vi "ATF_PUMP_PID_screen_V0.0.vi"() -> ()   [LabVIEW 2022 SP3]
panel:
  out "Countdown Timer (CDT)":dbl format="T%<+%H:%M:%S%3u>t"
  out "Date":timestamp format="%<%d/%m/%Y>T"
  in  "Close":bool
  in  "Screen No":dbl
  out "Indian Standard Time (IST)":timestamp format="%<%H:%M:%S%2u>T"
  out "B_AT_T_04":dbl format="%.2f bar"
  out "B_AT_T_05":dbl format="%.2f bar"
  out "B_ATP_P_01 76":dbl format="%.2f bar"
  out "B_ATP_P_01 75":dbl format="%.2f bar"
  out "B_ATP_P_01 74":dbl format="%.2f bar"
  out "B_ATP_P_01 73":dbl format="%.2f bar"
  out "B_ATP_P_01 72":dbl format="%.2f bar"
  out "B_ATP_P_01 71":dbl format="%.2f bar"
  out "B_ATP_P_01 70":dbl format="%.2f bar"
  out "B_ATP_P_01 69":dbl format="%.2f bar"
  out "B_ATP_P_01 68":dbl format="%.2f bar"
  out "B_ATP_P_01 67":dbl format="%.2f bar"
  out "B_ATP_P_01 66":dbl format="%.2f bar"
  out "B_ATP_P_01 65":dbl format="%.2f bar"
  out "B_ATP_P_01 64":dbl format="%.2f bar"
  out "B_ATP_P_01 63":dbl format="%.2f bar"
  out "B_ATP_P_01 62":dbl format="%.2f bar"
  out "B_ATP_P_01 61":dbl format="%.2f bar"
  out "B_ATP_P_01 60":dbl format="%.2f bar"
  out "B_ATP_P_01 59":dbl format="%.2f bar"
  out "B_ATP_P_01 58":dbl format="%.2f bar"
  out "B_ATP_P_01 57":dbl format="%.2f bar"
  out "B_ATP_P_01 56":dbl format="%.2f bar"
  out "B_ATP_P_01 55":dbl format="%.2f bar"
  out "B_ATP_P_01 54":dbl format="%.2f bar"
  out "B_ATP_P_01 53":dbl format="%.2f bar"
  out "B_ATP_P_01 52":dbl format="%.2f bar"
  out "B_ATP_P_01 51":dbl format="%.2f bar"
  out "B_ATP_P_01 50":dbl format="%.2f bar"
  out "B_ATP_P_01 49":dbl format="%.2f bar"
  out "B_ATP_P_01 48":dbl format="%.2f bar"
  out "B_ATP_P_01 47":dbl format="%.2f bar"
  out "B_ATP_P_01 46":dbl format="%.2f bar"
  out "B_ATP_P_01 45":dbl format="%.2f bar"
  out "B_ATP_P_01 44":dbl format="%.2f bar"
  out "B_ATP_P_01 43":dbl format="%.2f bar"
  out "B_ATP_P_01 42":dbl format="%.2f bar"
  out "B_ATP_P_01 41":dbl format="%.2f bar"
  out "B_ATP_P_01 40":dbl format="%.2f bar"
  out "B_ATP_P_01 39":dbl format="%.2f bar"
  out "B_ATP_P_01 38":dbl format="%.2f bar"
  out "B_ATP_P_01 37":dbl format="%.2f bar"
  out "B_ATP_P_01 36":dbl format="%.2f bar"
  out "B_ATP_P_01 35":dbl format="%.2f bar"
  out "B_ATP_P_01 34":dbl format="%.2f bar"
  out "B_ATP_P_01 33":dbl format="%.2f bar"
  out "B_ATP_P_01 32":dbl format="%.2f bar"
  out "B_ATP_P_01 31":dbl format="%.2f bar"
  out "B_ATP_P_01 30":dbl format="%.2f bar"
  out "B_ATP_P_01 29":dbl format="%.2f bar"
  out "B_ATP_P_01 28":dbl format="%.2f bar"
  out "B_ATP_P_01 27":dbl format="%.2f bar"
  out "B_ATP_P_01 26":dbl format="%.2f bar"
  out "B_ATP_P_01 25":dbl format="%.2f bar"
  out "B_ATP_P_01 24":dbl format="%.2f bar"
  out "B_ATP_P_01 23":dbl format="%.2f bar"
  out "B_ATP_P_01 22":dbl format="%.2f bar"
  out "B_ATP_P_01 21":dbl format="%.2f bar"
  out "B_ATP_P_01 20":dbl format="%.2f bar"
  out "B_ATP_P_01 19":dbl format="%.2f bar"
  out "B_ATP_P_01 18":dbl format="%.2f bar"
  out "B_ATP_P_01 17":dbl format="%.2f bar"
  out "B_ATP_P_01 16":dbl format="%.2f bar"
  out "B_ATP_P_01 15":dbl format="%.2f bar"
  out "B_ATP_P_01 14":dbl format="%.2f bar"
  out "B_ATP_P_01 13":dbl format="%.2f bar"
  out "B_ATP_P_01 12":dbl format="%.2f bar"
  out "B_ATP_P_01 11":dbl format="%.2f bar"
  out "B_ATP_P_01 10":dbl format="%.2f bar"
  out "B_ATP_P_01 9":dbl format="%.2f bar"
  out "B_ATP_P_01 8":dbl format="%.2f bar"
  out "B_ATP_P_01 7":dbl format="%.2f bar"
  out "B_ATP_P_01 6":dbl format="%.2f bar"
  out "B_ATP_P_01 5":dbl format="%.2f bar"
  out "B_ATP_P_01 4":dbl format="%.2f bar"
  out "B_ATP_P_01 3":dbl format="%.2f bar"
  out "B_ATP_P_01 2":dbl format="%.2f bar"
  out "B_ATP_P_01":dbl format="%.2f bar"
  out "B_LO_P_09":dbl format="%.2f bar"
  out "B_LO_P_10":dbl format="%.2f bar"
  out "B_AT_T_05":dbl format="%.2f bar"
  out "B_AT_T_04":dbl format="%.2f bar"
  out "B_LO_P_10":dbl format="%.2f bar"
  out "B_LO_P_09":dbl format="%.2f bar"
  # "BSTF P&ID SCREEN"
  # "VERSION 1.0"
  # "ATF MANIFOLD"
  # "ATF MANIFOLD"
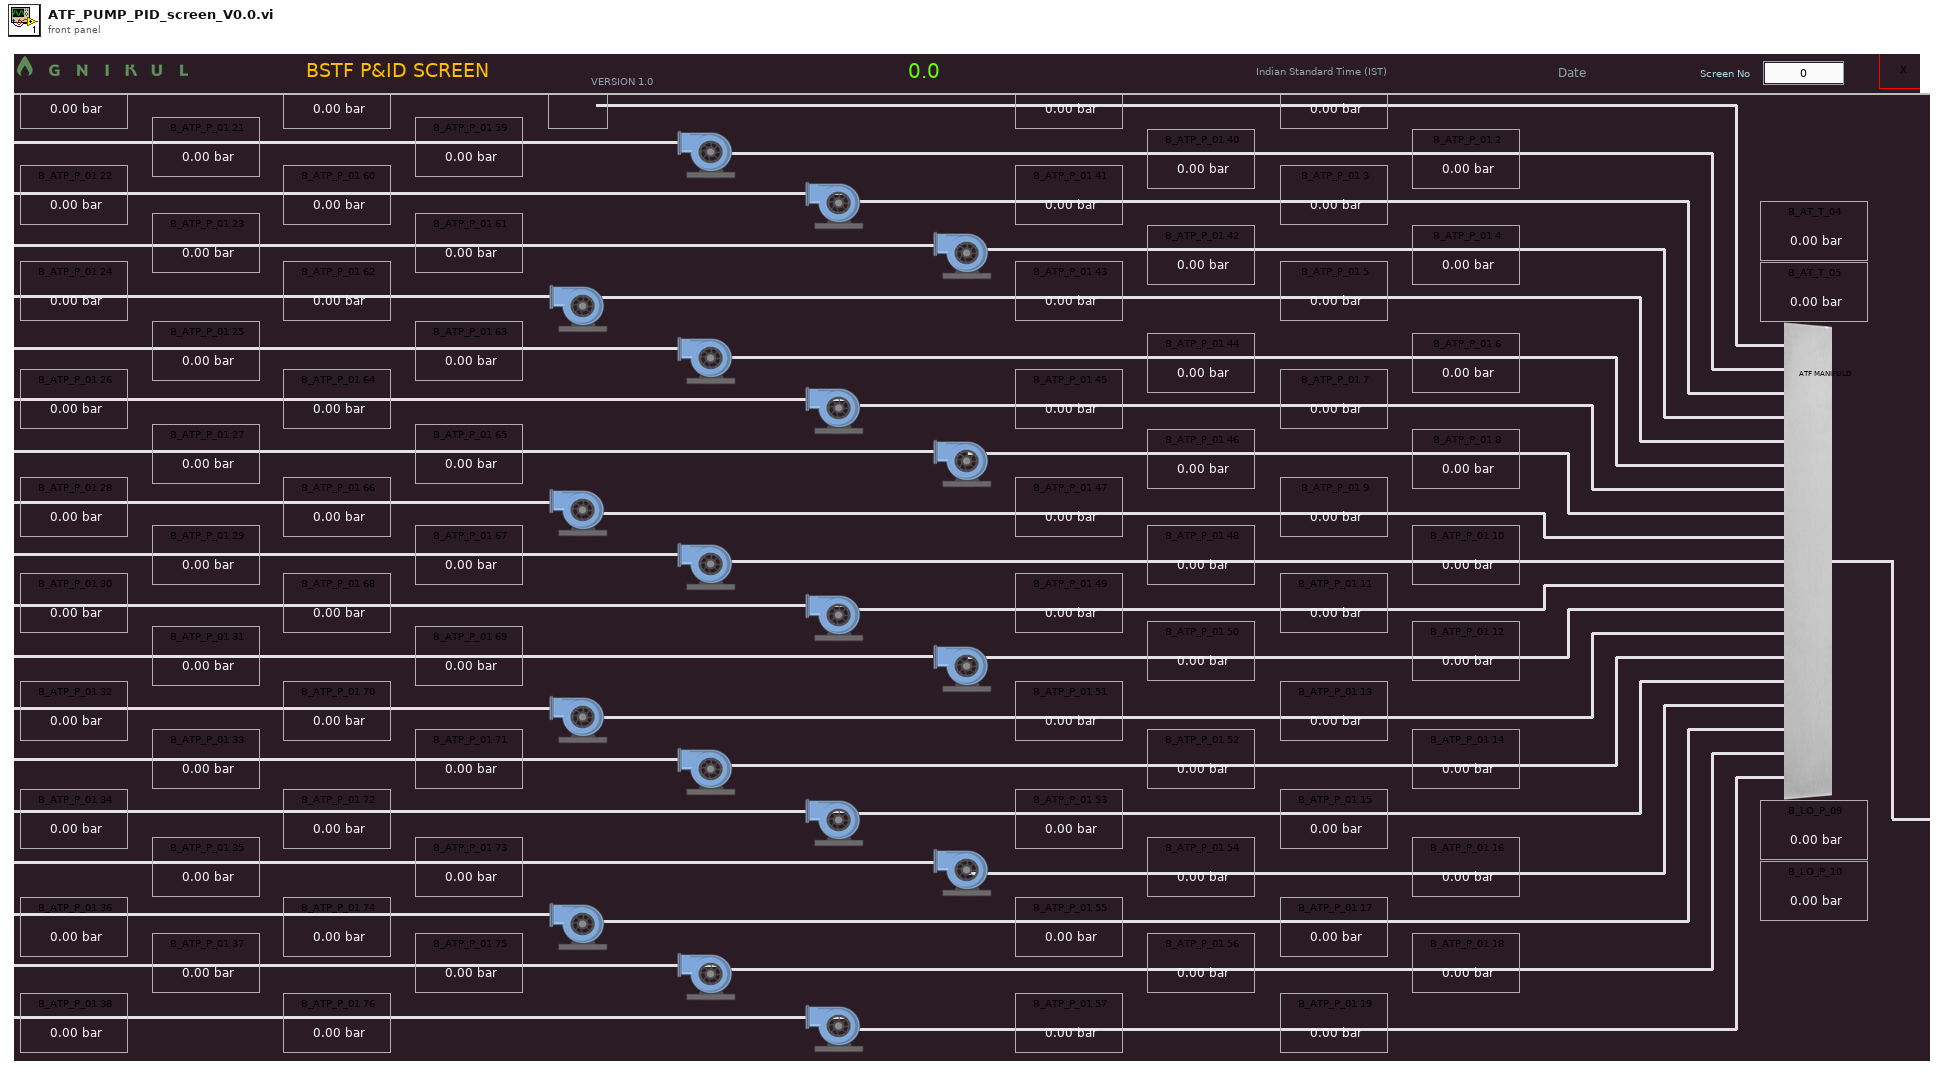
[diagram p1: front panel]
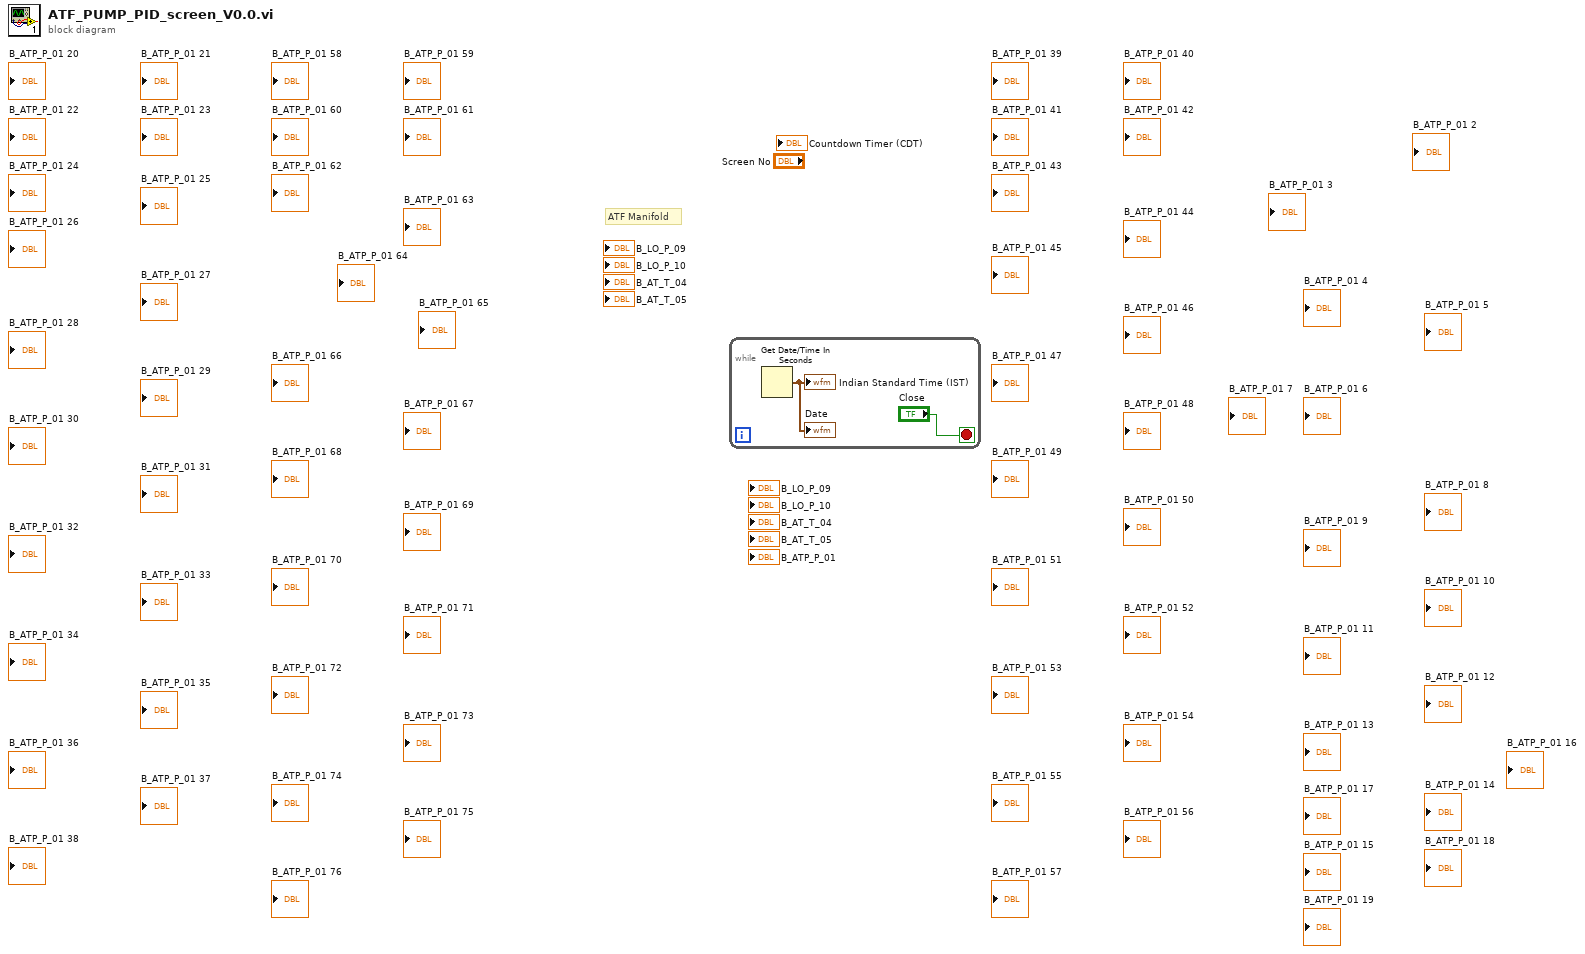
[diagram p0: block diagram]
diagram:
  # "ATF Manifold"
  n1 = while {
    stop <- "Close" stop-if-true
    n2 = Get Date/Time In Seconds() -> (seconds since 1Jan1904=→"Date" →"Indian Standard Time (IST)":timestamp)
  }
